vi "Dresden R2R Sputter 03.02.2018 IY24.vi"() -> ()   [LabVIEW 2009]
uses:
  ctl/Roll_StatusT.ctl
  <vilib>/Instr/_visa.llb/VISA Configure Serial Port (Instr).vi
  <vilib>/Utility/file.llb/Read From Spreadsheet File (string).vi
  <vilib>/NI Modbus.llb/MB Serial Master Query Read Discrete Inputs (poly).vi
  <vilib>/NI Modbus.llb/MB Serial Master Query Write Multiple Coils (poly).vi
  <vilib>/NI Modbus.llb/MB Serial Master Query Read Input Registers (poly).vi
  <vilib>/NI Modbus.llb/MB Serial Master Query Write Single Coil (poly).vi
  <vilib>/picture/picture.llb/Draw True-Color Pixmap.vi
panel:
  out "Actual Region led 5":bool
  out "Elapsed Time (s) 10":dbl caption="Elapsed Time (s)"
  in  "Right to Left 5":dbl=100000.0
  out "Elapsed Time (s) 9":dbl caption="Elapsed Time (s)"
  in  "Left to Right 5":dbl=100000.0
  out "Actual Region led 4":bool
  out "Elapsed Time (s) 8":dbl caption="Elapsed Time (s)"
  in  "Right to Left 4":dbl=100000.0
  out "Elapsed Time (s) 7":dbl caption="Elapsed Time (s)"
  in  "Left to Right 4":dbl=100000.0
  out "Actual Region led 3":bool
  out "Elapsed Time (s) 6":dbl caption="Elapsed Time (s)"
  in  "Right to Left 3":dbl=100000.0
  out "Elapsed Time (s) 5":dbl caption="Elapsed Time (s)"
  in  "Left to Right 3":dbl=100000.0
  in  "Speed":dbl=6.85 format="%.2g"
  in  "Roll_side_select":enum32{"Left to Right", "Right to Left"}(radio)=enum."Right to Left"
  in  "Parameters_set":bool
  in  "Calculate_auto":bool
  in  "Test_stop":bool
  in  "Start_roll":bool
  out "COM12 Loop Time":dbl caption="Present (s)" format="%.2f"
  in  "RPM":dbl=13.691
  out "Cevre":dbl
  out "Angle":dbl
  out "Gauge":dbl(knob) min=0.0 max=360.0 step=30.0 scale=0.0..360.0 scale format="%_2f"
  in  "Tension Parametre Set":bool
  out "Bacward Time":dbl
  out "Forward Time":dbl
  in  "Lap Count":i32=1
  in  "Cycle Sayisi":i32=1
  out "Current Chamber":i32=1
  out "Roll Status":T1
  out "Current Forward Lap":i32
  out "Current Cycle":i32
  out "Lap Times":dbl[](array[numeric])
  out "Current Backward Lap":i32
  in  "Moxa I/O 1":refnum<visa-resource-name>=refnum
  in  "Ch1_Motor_DO":bool
  in  "Ch3_Motor_DO":bool
  in  "Ch4_Motor_DO":bool
  in  "Ch2_Motor_DO":bool
  in  "Motor_Dir_DO":bool
  out "Ch1_Sensor_DI":bool
  out "Ch4_Sensor_DI":bool
  out "Ch2_Sensor_DI":bool
  out "Ch3_Sensor_DI":bool
  in  "Sensor_DI Sim":bool
  in  "Sim":bool
  in  "Ch1_3_2_do":bool
  in  "To Right Volt":dbl=6.85 format="%.2g"
  in  "To Left Volt":dbl=6.85 format="%.2g"
  out "COM12 Loop Time":dbl caption="Present (s)" format="%.2f"
  out "COM12 Time":dbl caption="Present (s)" format="%.2f"
  in  "Timer Reset Roll 2":bool
  in  "Left to Right":dbl=100000.0
  out "Elapsed Time (s) 2":dbl caption="Elapsed Time (s)"
  in  "Right to Left":dbl=100000.0
  out "Elapsed Time (s)":dbl
  out "Ch4_tab_led":bool
  out "Ch3_tab_led":bool
  out "Ch2_tab_led":bool
  out "Ch1_tab_led":bool
  in  "Start_Coating_MW":bool
  in  "Statue_abort":bool
  in  "Graph_tab_ch4":enum32{"Page 1"}(tab)
  out "Graph_pumping_time_ch4":dbl caption="Elapsed Time (s)" format="%<%H:%M:%S>t"
  out "Pressure_time_graph_ch4":dbl(graph)
  in  "Graph_tab_ch3":enum32{"Page 1"}(tab)
  out "Graph_pumping_time_ch3":dbl caption="Elapsed Time (s)" format="%<%H:%M:%S>t"
  out "Pressure_time_graph_ch3":dbl(graph)
  in  "Graph_tab_ch2":enum32{"Page 1"}(tab)
  out "Graph_pumping_time_ch2":dbl caption="Elapsed Time (s)" format="%<%H:%M:%S>t"
  out "Pressure_time_graph_ch2":dbl(graph)
  in  "MW_RF_Interlock":dbl=5e-05
  in  "Start_Coating_Ch4":bool
  in  "Single_ch3_Interlock":dbl=5e-05
  in  "MW_Coating_Interlock 6":dbl=5e-05
  in  "Start_Coating_Ch3":bool
  in  "Start_Coating_Ch2":bool
  in  "Single_Ch2_Interlock":dbl=5e-05
  in  "MW_Coating_Interlock 5":dbl=5e-05
  in  "R General_tab":enum32{"Page 1", "Page 2"}(tab)
  in  "R_Cancel":bool caption="Cancel"
  in  "Thickness_Monitor_Active":bool
  in  "Recipe_selection tab":T2(tab)
  in  "R_Simple_Coating Type Selection":T3(radio)
  in  "R_Single_Coating Type Selection_tab":T4(tab)
  in  "R_Single Microwave Time":dbl caption="sec"
  in  "R_Single Microwave Power":dbl caption="Watt"
  in  "R Single Microwave Number":dbl
  in  "R_DC_Chamber_selection":enum32{"Chamber II", "Chamber III"}(radio)
  in  "R Single DC Interval length":dbl
  in  "R Single DC Step5 Coating Power Active":bool
  in  "R Single DC Step5 Coating Power":dbl caption="Watt"
  in  "R Single DC Step4 Coating Power Active":bool
  in  "R Single DC Step4 Coating Power":dbl caption="Watt"
  in  "R Single DC Step3 Coating Power Active":bool
  in  "R Single DC Step3 Coating Power":dbl caption="Watt"
  in  "R Single DC Step2 Coating Power Active":bool
  in  "R Single DC Step2 Coating Power":dbl caption="Watt"
  in  "R Single DC Step1 Coating Power Active":bool
  in  "R Single DC Step1 Coating Power":dbl caption="Watt"
  in  "R_Single DC_Material ok":bool
  in  "R_Single DC_Mat_sel":u64(ring) items=["Other", "Ag", "AgBr", "AgCl", "Al", "Al2O3", "As", "Au", "B", "Ba", "Be", "Bi", "Bi2O3", "C (Diamond)", "C (Graphite)", "Ca", "CaF", "Cd", "CdS", "CdSe", "CdTe", "CeF3", "CeO", "Cr", "Cr2O3", "Co", "Cu", "Cu2S (A)", "Cu2S (B)", "CuS", "Dy", "Er", "Fe", "Ga", "GaAs", "Gd", "Ge", "Hf", "HfO2", "Hg", "Ho", "In", "InSb", "In2O3", "Ir", "KCl", "La", "LaF3", "LaO3", "Li", "LiF", "Mg", "MgF2", "MgO", "Mn", "MnS", "Mo", "Na", "NaCl", "NdF3", "Nd2O3", "Ni", "Nb", "Nb2O5", "Pb", "PbS", "Pd", "Pt", "Re", "Rh", "Rb", "S", "Sb", "Sc", "Se", "Si", "SiO", "SiO2", "Sm", "Sn", "Ta", "Ta2O5", "Te", "Tb", "ThF4", "Ti", "TiO2", "TiO", "Tl", "U", "V", "W", "WC", "Y", "Y2O3", "Yb", "Zn", "ZnO", "ZnSe", "ZnS", "Zr", "ZrO2", "Si3N4", "ITO", "PbI2"]
  in  "R Single DC Target material":string
  in  "R Single DC Ignition Power":dbl caption="Watt"
  in  "R Single DC Target Clean":bool
  in  "R Single DC Target Clean Time":dbl caption="min" format="%.1f"
  in  "R Single DC Target Clean Power":dbl caption="Watt"
  in  "R Single RF Interval length":dbl
  in  "R Single RF Step5 Coating Power Active":bool
  in  "R Single RF Step5 Coating Power":dbl caption="Watt"
  in  "R Single RF Step4 Coating Power Active":bool
  in  "R Single RF Step4 Coating Power":dbl caption="Watt"
  in  "R Single RF Step3 Coating Power Active":bool
  in  "R Single RF Step3 Coating Power":dbl caption="Watt"
  in  "R Single RF Step2 Coating Power Active":bool
  in  "R Single RF Step2 Coating Power":dbl caption="Watt"
  in  "R Single RF Step1 Coating Power Active":bool
  in  "R_Single RF Material ok":bool
  in  "R_Single RF_Mat_sel":u64(ring) items=["Other", "Ag", "AgBr", "AgCl", "Al", "Al2O3", "As", "Au", "B", "Ba", "Be", "Bi", "Bi2O3", "C (Diamond)", "C (Graphite)", "Ca", "CaF", "Cd", "CdS", "CdSe", "CdTe", "CeF3", "CeO", "Cr", "Cr2O3", "Co", "Cu", "Cu2S (A)", "Cu2S (B)", "CuS", "Dy", "Er", "Fe", "Ga", "GaAs", "Gd", "Ge", "Hf", "HfO2", "Hg", "Ho", "In", "InSb", "In2O3", "Ir", "KCl", "La", "LaF3", "LaO3", "Li", "LiF", "Mg", "MgF2", "MgO", "Mn", "MnS", "Mo", "Na", "NaCl", "NdF3", "Nd2O3", "Ni", "Nb", "Nb2O5", "Pb", "PbS", "Pd", "Pt", "Re", "Rh", "Rb", "S", "Sb", "Sc", "Se", "Si", "SiO", "SiO2", "Sm", "Sn", "Ta", "Ta2O5", "Te", "Tb", "ThF4", "Ti", "TiO2", "TiO", "Tl", "U", "V", "W", "WC", "Y", "Y2O3", "Yb", "Zn", "ZnO", "ZnSe", "ZnS", "Zr", "ZrO2", "Si3N4", "ITO", "PbI2"]
  in  "R Single RF Target material":string
  in  "R Single RF Ignition Power":dbl caption="Watt"
  in  "R Single RF Target Clean Power":dbl caption="Watt"
  in  "R Single RF Target Clean Time":dbl caption="min" format="%.1f"
  in  "R Single RF Target Clean":bool
  in  "R Single RF Ramp down":bool
  in  "R Single RF Ramp down Time":dbl caption="sec"
  in  "R Single RF  Step1 Coating Power":dbl caption="Watt"
  in  "R Single RF Ramp up Time":dbl caption="sec"
  in  "R Single RF Ramp up":bool
  in  "R Cmb Interval length":dbl
  in  "R Cmb Ch2 DC Target Clean Power Active":bool
  in  "R Cmb Ch3 Step5 Coating Power":dbl caption="Watt"
  in  "R Cmb Ch3 Step4 Coating Power":dbl caption="Watt"
  in  "R Cmb Ch3 Step3 Coating Power":dbl caption="Watt"
  in  "R Cmb Ch3 Step2 Coating Power":dbl caption="Watt"
  in  "R Cmb Ch3 Step1 Coating Power":dbl caption="Watt"
  in  "R Cmb Ch2 Step5 Coating Power Active":bool
  in  "R Cmb Ch2 Step5 Coating Power":dbl caption="Watt"
  in  "R Cmb Ch2 Step4 Coating Power Active":bool
  in  "R Cmb Ch2 Step4 Coating Power":dbl caption="Watt"
  in  "R Cmb Ch2 Step3 Coating Power Active":bool
  in  "R Cmb Ch2 Step3 Coating Power":dbl caption="Watt"
  in  "R Cmb Ch2 Step2 Coating Power Active":bool
  in  "R Cmb Ch2 Step2 Coating Power":dbl caption="Watt"
  in  "R Cmb Ch2 Step1 Coating Power Active":bool
  in  "R Cmb Ch2 Step1 Coating Power":dbl caption="Watt"
  in  "R Cmb Ch3 Material ok":bool
  in  "R Cmb Ch3 Mat_sel":u64(ring) items=["Other", "Ag", "AgBr", "AgCl", "Al", "Al2O3", "As", "Au", "B", "Ba", "Be", "Bi", "Bi2O3", "C (Diamond)", "C (Graphite)", "Ca", "CaF", "Cd", "CdS", "CdSe", "CdTe", "CeF3", "CeO", "Cr", "Cr2O3", "Co", "Cu", "Cu2S (A)", "Cu2S (B)", "CuS", "Dy", "Er", "Fe", "Ga", "GaAs", "Gd", "Ge", "Hf", "HfO2", "Hg", "Ho", "In", "InSb", "In2O3", "Ir", "KCl", "La", "LaF3", "LaO3", "Li", "LiF", "Mg", "MgF2", "MgO", "Mn", "MnS", "Mo", "Na", "NaCl", "NdF3", "Nd2O3", "Ni", "Nb", "Nb2O5", "Pb", "PbS", "Pd", "Pt", "Re", "Rh", "Rb", "S", "Sb", "Sc", "Se", "Si", "SiO", "SiO2", "Sm", "Sn", "Ta", "Ta2O5", "Te", "Tb", "ThF4", "Ti", "TiO2", "TiO", "Tl", "U", "V", "W", "WC", "Y", "Y2O3", "Yb", "Zn", "ZnO", "ZnSe", "ZnS", "Zr", "ZrO2", "Si3N4", "ITO", "PbI2"]
  in  "R Cmb Ch3 Target material":string
  in  "R Cmb Ch3 DC Ignition Power":dbl caption="Watt"
  in  "R Cmb Ch3 DC Target Clean Power Active":bool
  in  "R Cmb Ch3 DC Target Clean Time":dbl caption="min" format="%.1f"
  in  "R Cmb Ch3 DC Target Clean Power":dbl caption="Watt"
  in  "R_Cmb Ch2_Material ok":bool
  in  "R_Cmb Ch2_Mat_sel":u64(ring) items=["Other", "Ag", "AgBr", "AgCl", "Al", "Al2O3", "As", "Au", "B", "Ba", "Be", "Bi", "Bi2O3", "C (Diamond)", "C (Graphite)", "Ca", "CaF", "Cd", "CdS", "CdSe", "CdTe", "CeF3", "CeO", "Cr", "Cr2O3", "Co", "Cu", "Cu2S (A)", "Cu2S (B)", "CuS", "Dy", "Er", "Fe", "Ga", "GaAs", "Gd", "Ge", "Hf", "HfO2", "Hg", "Ho", "In", "InSb", "In2O3", "Ir", "KCl", "La", "LaF3", "LaO3", "Li", "LiF", "Mg", "MgF2", "MgO", "Mn", "MnS", "Mo", "Na", "NaCl", "NdF3", "Nd2O3", "Ni", "Nb", "Nb2O5", "Pb", "PbS", "Pd", "Pt", "Re", "Rh", "Rb", "S", "Sb", "Sc", "Se", "Si", "SiO", "SiO2", "Sm", "Sn", "Ta", "Ta2O5", "Te", "Tb", "ThF4", "Ti", "TiO2", "TiO", "Tl", "U", "V", "W", "WC", "Y", "Y2O3", "Yb", "Zn", "ZnO", "ZnSe", "ZnS", "Zr", "ZrO2", "Si3N4", "ITO", "PbI2"]
  in  "R Cmb Ch2 Target material":string
  in  "R Cmb Ch2 DC Ignition Power":dbl caption="Watt"
  in  "R Cmb Ch2 DC Target Clean Time":dbl caption="min" format="%.1f"
  in  "R Cmb Ch2 DC Target Clean Power":dbl caption="Watt"
  in  "R Cmb Number of pairs":dbl
  in  "Substrate Material":string
  in  "Recipe Name":string
  in  "R_Recipe_type_selection":enum32{"Single Recipe", "Combination Sputter"}(radio)
  in  "R_Web_selection":enum32{"Web", "Other"}(radio)=enum."Other"
  in  "Web_selection_tab":T5(tab)
  in  "R Web thicness":dbl
  in  "R Maximum diameter":dbl format="%.1f"
  in  "R Minimum diameter":dbl
  in  "R Web speed(cm/min)":dbl
  in  "R Tension Value":dbl
  out "R _Total_length":dbl caption="m" format="%.1f"
  in  "R_Calculate":bool
  in  "R_Thickness Selection":enum32{"Thickness", "Time"}(radio)
  in  "R_Target Thickness Value":dbl format="%.2f"
  in  "R_Duration":dbl caption="%"
  in  "R Set Pressure mtorr":dbl caption="mTorr" format="%.1f"
  in  "R Argon Flow sccm":dbl caption="sccm"
  in  "R Z_factor":dbl format="%_3f"
  in  "R Material_density":dbl caption="g/cm3" format="%_3f"
  in  "R_OK":bool caption="OK2"
  in  "R Toooling_factor":dbl caption="%"
  in  "Clear_error":bool
  in  "Gv_tab_ch2_3_gui":enum32{"Page 1", "Page 2"}(tab)
  in  "Gv_open ch2_3_gui":bool
  in  "Gv_close_ch2_3_gui":bool
  out "Error Message":string
  out "Process_flow":string
  in  "MOUSE":enum32{"Page 1", "Page 2", "Page 3", "Page 4"}(tab)=enum."Page 4"
  out "Mouse Position":cluster{"X":i32, "Y":i32}
  out "Mouse Position 3":cluster{"X":i32, "Y":i32}
  out "Mouse Position 5":cluster{"X":i32, "Y":i32}
  out "Mouse Position 4":cluster{"X":i32, "Y":i32}
  out "Mouse Position 2":cluster{"X":i32, "Y":i32}
  out "Mouse Position 8":cluster{"X":i32, "Y":i32}
  out "Mouse Position 7":cluster{"X":i32, "Y":i32}
  out "Mouse Position 6":cluster{"X":i32, "Y":i32}
  out "Mouse Position 9":cluster{"X":i32, "Y":i32}
  in  "general tab":T6(tab)
  out "DESCRIPTION":string
  in  "Graph_tab_ch1":enum32{"Page 1"}(tab)
  out "Graph_pumping_time_ch1":dbl caption="Elapsed Time (s)" format="%<%H:%M:%S>t"
  out "Pressure_time_graph_ch1":dbl(graph)
  out "Pressure_gui":dbl format="%.1f"
  out "Ch_CC_press_ch1_gui1":dbl format="%#_2e"
  out "Ch_pg_press_ch1_gui":dbl caption="Torr" format="%#_2e"
  out "Pl_pg_press_ch1_gui":dbl caption="Torr" format="%#_2e"
  out "Ch_CC_press_ch2":dbl format="%_2e"
  out "Ch_pg_press_ch2_gui":dbl caption="Torr" format="%#_2e"
  out "Pressure 2_gui":i32 format="%.1f"
  in  "Pl_vbv_ch3_tab_gui":enum32{"Page 1", "Page 2"}(tab)
  in  "Ch3_Pl_vbv_stop_gui":bool
  in  "Ch3_Pl_vbv_start_gui":bool
  in  "Pl_vbv_ch2_tab_gui":enum32{"Page 1", "Page 2"}(tab)
  in  "Ch2_Pl_vbv_stop_gui":bool
  in  "Ch2_Pl_vbv_start_gui":bool
  in  "Mp_ch3_tab_gui":enum32{"Page 1", "Page 2"}(tab)
  in  "Ch3_Mp_stop_gui":bool
  in  "Ch3_Mp_start_gui":bool
  in  "Mp_ch2_tab_gui":enum32{"Page 1", "Page 2"}(tab)
  in  "Ch2_Mp_stop_gui":bool
  in  "Ch2_Mp_start_gui":bool
  in  "Gv_tab_ch1_2_gui":enum32{"Page 1", "Page 2"}(tab)
  in  "Gv_close_ch1_2_gui":bool
  in  "Gv_open ch1_2_gui":bool
  in  "Gv_tab_ch3_4gui":enum32{"Page 1", "Page 2"}(tab)
  in  "Gv_close_ch3_4gui":bool
  in  "Gv_open ch3_4gui":bool
  in  "Pc_bv_tab_ch3_gui":enum32{"Page 1", "Page 2"}(tab)
  in  "Pc_bv_close_ch3_gui":bool
  in  "Pc_bv_open_ch3_gui":bool
  in  "Pc_bv_tab_ch2_gui":enum32{"Page 1", "Page 2"}(tab)
  in  "Pc_bv_close_ch2_gui":bool
  in  "Pc_bv_open_ch2_gui":bool
  in  "Pc_bv_tab_ch4_gui":enum32{"Page 1", "Page 2"}(tab)
  in  "Pc_bv_close_ch4_gui":bool
  in  "Pc_bv_open_ch4_gui":bool
  in  "Pc_bv_tab_ch1_gui":enum32{"Page 1", "Page 2"}(tab)
  in  "Pc_bv_close_ch1_gui":bool
  in  "Pc_bv_open_ch1_gui":bool
  in  "Trns_gv_bp_ch2_gui":enum32{"Page 1", "Page 2"}(tab)
  in  "Ch2_Trns_gv_bp_close_gui":bool
  in  "Ch2_Trns_gv_bp_open_gui":bool
  in  "Trns_gv_bp_ch3_gui":enum32{"Page 1", "Page 2"}(tab)
  in  "Ch3_Trns_gv_bp_close_gui":bool
  in  "Ch3_Trns_gv_bp_open_gui":bool
  in  "Trns_gv_bp2_ch2_gui":enum32{"Page 1", "Page 2"}(tab)
  in  "Ch2_Trns_gv_bp2_close_gui":bool
  in  "Ch2_Trns_gv_bp2_open_gui":bool
  in  "Trns_gv_bp2_ch3_gui":enum32{"Page 1", "Page 2"}(tab)
  in  "Ch3_Trns_gv_bp2_close_gui":bool
  in  "Ch3_Trns_gv_bp2_open_gui":bool
  in  "Tp_ch3_tab_gui":enum32{"Page 1", "Page 2"}(tab)
  in  "Tp_stop_ch3_gui":bool
  in  "Tp_start_ch3_gui":bool
  in  "Tp_ch2_tab_gui":enum32{"Page 1", "Page 2"}(tab)
  in  "Tp_stop_ch2_gui":bool
  in  "Tp_start_ch2_gui":bool
  in  "Tp_ch4_tab_gui":enum32{"Page 1", "Page 2"}(tab)
  in  "Tp_stop_ch4_gui":bool
  in  "Tp_start_ch4_gui":bool
  in  "Tp_ch1_tab_gui":enum32{"Page 1", "Page 2"}(tab)
  in  "Tp_stop_ch1_gui":bool
  in  "Tp_start_ch1_gui":bool
  in  "Ch_vbv_tab_ch3_gui":enum32{"Page 1", "Page 2"}(tab)
  in  "Ch3_Ch_vbv_close_gui":bool
  in  "Ch3_Ch_vbv_open_gui":bool
  in  "Ch_vbv_tab_ch2_gui":enum32{"Page 1", "Page 2"}(tab)
  in  "Ch2_Ch_vbv_close_gui":bool
  in  "Ch2_Ch_vbv_open_gui":bool
  in  "Ch_vbv_tab_ch4_gui":enum32{"Page 1", "Page 2"}(tab)
  in  "Ch4_Ch_vbv_close_gui":bool
  in  "Ch4_Ch_vbv_open_gui":bool
  in  "Ch_vbv_tab_ch1_gui":enum32{"Page 1", "Page 2"}(tab)
  in  "Ch1_Ch_vbv_close_gui":bool
  in  "Ch1_Ch_vbv_open_gui":bool
  in  "Tp_bv_tab_ch3_gui":enum32{"Page 1", "Page 2"}(tab)
  in  "Ch3_Tp_bv_close_gui":bool
  in  "Ch3_Tp_bv_open_gui":bool
  in  "Tp_bv_tab_ch2_gui":enum32{"Page 1", "Page 2"}(tab)
  in  "Ch2_Tp_bv_close_gui":bool
  in  "Ch2_Tp_bv_open_gui":bool
  in  "Tp_bv_tab_ch4_gui":enum32{"Page 1", "Page 2"}(tab)
  in  "Ch4_Tp_bv_close_gui":bool
  in  "Ch4_Tp_bv_open_gui":bool
  in  "Tp_bv_tab_ch1_gui":enum32{"Page 1", "Page 2"}(tab)
  in  "Ch1_Tp_bv_close_gui":bool
  in  "Ch1_Tp_bv_open_gui":bool
  in  "Pl_vbv_tab_ch1_gui":enum32{"Page 1", "Page 2"}(tab)
  in  "Ch1_Pl_vbv_close_gui":bool
  in  "Ch1_Pl_vbv_open_gui":bool
  in  "Pl_vbv_ch4_tab_gui":enum32{"Page 1", "Page 2"}(tab)
  in  "Ch4_Pl_vbv_stop_gui":bool
  in  "Ch4_Pl_vbv_start_gui":bool
  in  "Mp_ch4_tab_gui":enum32{"Page 1", "Page 2"}(tab)
  in  "Ch4_Mp_stop_gui":bool
  in  "Ch4_Mp_start_gui":bool
  in  "Mp_ch1tab_gui":enum32{"Page 1", "Page 2"}(tab)
  ... 2784 more
  # "CHAMBER 4"
  # "CHAMBER 3"
  # "CHAMBER 2"
  # "CHAMBER 1"
  # "Load Coating and Automatic Coating"
  # "Load Coating and Automatic Coating"
  # "Load Coating and Automatic Coating"
  # "PROCESS FLOW"
  # "ERROR MESSAGE"
  # "Chamber Pressure"
  # "Torr"
  # "Automatic Pumping Time"
  # "Chamber Pressure"
  # "Torr"
  # "Automatic Pumping Time"
  # "Chamber Pressure"
  # "Torr"
  # "Automatic Pumping Time"
  # "Coating Interlock :"
  # "Single Coating Interlock            :"
  # "Combination Coating Interlock  :"
  # "Single Coating Interlock             :"
  # "Combination Coating Interlock  :"
  # "Recipe  Selection"
  # "Web  Selection"
  # "Thickness Monitor Parameters"
  # "Pressure Control Parameters"
  # "Material Density       :"
  # "Argon Flow         :"
  # "Z factor                    :"
  # "Set Pressure        :"
  # "Tooling Factor         :"
  # "Coating Type Selction"
  # "Power Value :"
  # "Watt"
  # "Duration      :"
  # "sec"
  # "Times          :"
  # "DCPS Parameters"
  # "Target material          :"
  # "Ignition Power           :"
  # "Target Clean Power    :"
  # "Interval length:"
  # "m"
  # "Coating Power  Step 1:"
  # "Coating Power  Step 2:"
  # "Coating Power  Step 3:"
  # "Coating Power  Step 4:"
  # "Coating Power  Step 5:"
  # "RFPS Parameters"
  # "Target material          :"
  # "Ramp Up Time           :"
  # "Ignition Power           :"
  # "Target Clean Power    :"
  # "Coating Power  Step 1:"
  # "Interval length:"
  # "m"
  # "Coating Power  Step 2:"
  # "Coating Power  Step 3:"
  # "Coating Power  Step 4:"
  # "Coating Power  Step 5:"
  # "Ramp Down Time      :"
  # "DCPS Parameters"
  # "CHAMBER II"
  # "CHAMBER III"
  # "Target material          :"
  # "Target material         :"
  # "Ignition Power           :"
  # "Ignition Power          :"
  # "Target Clean Power    :"
  # "Target Clean Power   :"
  # "Coating Power  Step 1:"
  # "Coating Power  Step 2:"
  # "Coating Power  Step 3:"
  # "Coating Power  Step 4:"
  # "Coating Power  Step 5:"
  # "Interval length:"
  # "m"
  # "Number of pair:"
  # "Roll  Parameters"
  # "Minimum Diameter      :"
  # "mm"
  # "Web Speed              :"
  # "cm / min"
  # "Tension Value         :"
  # "Maximum Diameter     :"
  # "mm"
  # "N"
  # "Web Thickness            :"
  # "µm"
  # "Total Length           :"
  # "Other Parameters"
  # "Thickness Selection         :"
  # "Target Thickness Value   :"
  # "kA"
  # "sec"
  # "Hz"
  # "Hz"
  # "Hz"
  # "Hz"
  # "CH 4"
  # "CH 3"
  # "CH 2"
  # "CH 1"
  # "Torr"
  # "Torr"
  # "Torr"
  # "Torr"
  # "Torr"
  # "mTorr"
  # "mTorr"
  # "mTorr"
  # "mTorr"
  # "mTorr"
  # "DESCRIPTION"
  # "Chamber Pressure"
  # "Torr"
  # "Automatic Pumping Time"
  # "CHAMBER 4"
  # "CHAMBER 2"
  # "CHAMBER 3"
  # "CHAMBER 1"
  # "Valve Control"
  # "Chamber Pressure"
  # "Torr"
  # "Target Pressure"
  # "Torr"
  # "Hour"
  # "Automatic Pumping Time"
  # "TP-BV"
  # "BG-BV"
  # "TRNS -GV-BP"
  # "PC-BV"
  # "Vacuum Pump Control"
  # "Vacuum Break Valve Control"
  # "PL-VBV"
  # "MP"
  # "TP"
  # "CH-VBV"
  # "Turbo Pump Settings"
  # "Low Speed"
  # "Hz"
  # "Tp Status"
  # "P vs t Graph"
  # "Air pressure check"
  # "CH-ATM close"
  # "Chamber Door check"
  # "PL-ATM close"
  # "Center WFS check"
  # "MP start"
  # "WFC  check"
  # "Pipe Line pressure  check"
  # "TRNS-GV close  check"
  # "Chamber pressure  check"
  # "TP stop"
  # "BG-BV  open"
  # "CC close"
  # "Chamber pressure  check"
  # "BG-BV close"
  # "TP  start"
  # "TP-BV close"
  # "Chamber pressure check"
  # "PL-ATM false"
  # "CC  open"
  # "MP stop"
  # "Trns-GV-BP close"
  # "PL-VBV open"
  # "Target Pressure reach"
  # "Pipe Line pressure check"
  # "Automatic  Vacuum Pumping finish"
  # "CH-ATM false"
  # "PC-BV open"
  # "CH-VBV  open"
  # "Trns-GV-BP open/close"
  # "CH-ATM check"
  # "CH-VBV close"
  # "PL-VBV close"
  # "TP-BV open"
  # "Air pressure check"
  # "Chamber Door check"
  # "Center WFS check"
  # "WFC check"
  # "Trns GV close  check"
  # "CH-VBV close"
  # "PL-VBV close"
  # "CH-ATM close"
  # "PL-ATM close"
  # "MP start"
  # "Pipe line pressure  dropped to below 0.9 Torr"
  # "Chamber pressure  dropped to below 0.9 Torr"
  # "TP-BV open"
  # "PC-BV open"
  # "Trns GV-BP  open/close"
  # "Chamber pressure   dropped to below 0.9   Torr"
  # "BG-BV open"
  # "Chamber pressure   dropped to below 0.9   Torr"
  # "TP start"
  # "CC open"
  # "Trns-GV-BP close"
  # "Target Pressure Value reach"
  # "Automatic  Vacuum Pumping finish"
  # "Waiting Tp speed drop to  800 Hz"
  # "CC close"
  # "BG-BV close"
  # "PC-BV close"
  # "PC-BV  open if vacuum break."
  # "TP-BV close"
  # "MP stop"
  # "PL-VBV open"
  # "PL-VBV close"
  # "Waiting Tp speed drop to  730 Hz"
  # "CH-VBV open if vacuum break"
  # "CH-VBV close if vacuum break"
  # "CH-VBV open if vacuum break"
  # "TRNS-GV-BP  open if vacuum break"
  # "CH-ATM check if vacuum break"
  # "TRNS-GV-BP  close"
  # "CH-VBV close if vacuum break"
  # "PC-BV close if vacuum break"
  # "CH-VBV check"
  # "Shutdown process finish"
  # "Vacuum Break Valve Control"
  # "Vacuum Pump Control"
  # "Chamber Pressure"
  # "Torr"
  # "Target Pressure"
  # "Torr"
  # "Hour"
  # "Automatic Pumping Time"
  # "Valve Control"
  # "BG-BV"
  # "TP-BV"
  # "TRNS -GV-BP"
  # "TRNS -GV-BP2"
  # "PC-BV"
  # "TP"
  # "PL-VBV"
  # "MP"
  # "CH-VBV"
  # "Turbo Pump Settings"
  # "Low Speed"
  # "Hz"
  # "Tp Status"
  # "P vs t Graph"
  # "Air pressure check"
  # "TP-BV open"
  # "Chamber Door check"
  # "CH-ATM close"
  # "Center WFS check"
  # "PL-ATM close"
  # "WFC  check"
  # "MP start"
  # "TRNS-GV 2_3_close  check"
  # "Pipe Line pressure  check"
  # "Chamber pressure  check"
  # "TRNS-GV 3_ 4close  check"
  # "TP stop"
  # "BG-BV  open"
  # "Chamber pressure  check"
  # "CC close"
  # "TP  start"
  # "BG-BV close"
  # "TP-BV close"
  # "Chamber pressure check"
  # "PL-ATM false"
  # "CC  open"
  # "Trns-GV-BP close"
  # "MP stop"
  # "Trns-GV-BP2 close"
  # "PL-VBV open"
  # "Target Pressure reach"
  # "Pipe Line pressure check"
  # "CH-ATM false"
  # "Automatic  Vacuum Pumping finish"
  # "PC-BV open"
  # "CH-VBV  open"
  # "Trns-GV-BP2 open/close"
  # "Trns-GV-BP open/close"
  # "CH-ATM check"
  # "CH-VBV close"
  # "PL-VBV close"
  # "Air pressure check"
  # "Chamber Door check"
  # "Center WFS check"
  # "WFC check"
  # "Trns GV_2_3 close  check"
  # "Trns GV_3_4close  check"
  # "CH-VBV close"
  # "PL-VBV close"
  # "CH-ATM close"
  # "PL-ATM close"
  # "MP start"
  # "Pipe line pressure  dropped to below 0.9 Torr"
  # "Chamber pressure  dropped to below 0.9 Torr"
  # "TP-BV open"
  # "PC-BV open"
  # "Trns GV-BP2  open/close"
  # "Trns GV-BP  open/close"
  # "Chamber pressure   dropped to below 0.9   Torr."
  # "BG-BV open"
  # "Chamber pressure   dropped to below 0.9   Torr"
  # "TP2 start"
  # "CC open"
  # "Trns-GV-BP close"
  # "Trns-GV-BP2 close"
  # "Target Pressure Value reach"
  # "Automatic  Vacuum Pumping finish"
  # "Waiting Tp speed drop to  800 Hz"
  # "CC close"
  # "BG-BV close"
  # "PC-BV close"
  # "PC-BV  open if vacuum break."
  # "TP-BV close"
  # "MP stop"
  # "PL-VBV open"
  # "PL-VBV close"
  # "Waiting Tp speed drop to  730 Hz if vacuum break"
  # "CH-VBV open if vacuum break"
  # "CH-VBV close if vacuum break"
  # "CH-VBV open if vacuum break"
  # "TRNS-GV-BP 2 open if vacuum break"
  # "TRNS-GV-BP  open if vacuum break"
  # "CH-ATM check if vacuum break"
  # "TRNS-GV-BP 2 close"
  # "TRNS-GV-BP close"
  # "CH-VBV close if vacuum break"
  # "PC-BV close if vacuum break"
  # "CH-VBV check"
  # "Shutdown process finish"
  # "Valve Control"
  # "Vacuum Break Valve Control"
  # "Vacuum Pump Control"
  # "Chamber Pressure"
  # "Torr"
  # "Target Pressure"
  # "Torr"
  # "Hour"
  # "Automatic Pumping Time"
  # "BG-BV"
  # "TP-BV"
  # "TRNS -GV-BP2"
  # "TRNS -GV-BP"
  # "PC-BV"
  # "TP"
  # "MP"
  # "PL-VBV"
  # "CH-VBV"
  # "Turbo Pump Settings"
  # "Low Speed"
  # "Hz"
  # "Tp Status"
  # "P vs t Graph"
  # "PL-ATM close"
  # "Air pressure check"
  # "MP start"
  # "Chamber Door check"
  # "Pipe Line pressure  check"
  # "Center WFS check"
  # "Chamber pressure  check"
  # "WFC  check"
  # "BG-BV  open"
  # "TRNS-GV 1_2_close  check"
  # "Chamber pressure  check"
  # "TRNS-GV 2_ 3close  check"
  # "TP  start"
  # "TP stop"
  # "Chamber pressure check"
  # "CC close"
  # "CC  open"
  # "BG-BV close"
  # "Trns-GV-BP close"
  # "TP-BV close"
  # "Trns-GV-BP2 close"
  # "PL-ATM false"
  # "Target Pressure reach"
  # "MP stop"
  # "Automatic  Vacuum Pumping finish"
  # "PL-VBV open"
  # "Pipe Line pressure check"
  # "CH-ATM false"
  # "PC-BV open"
  # "CH-VBV  open"
  # "Trns-GV-BP2 open/close"
  # "Trns-GV-BP open/close"
  # "CH-ATM check"
  # "CH-VBV close"
  # "PL-VBV close"
  # "TP-BV open"
  # "CH-ATM close"
  # "Air pressure check"
  # "Chamber Door check"
  # "Center WFS check"
  # "WFC check"
  # "Trns GV close  check"
  # "Trns GV close  check"
  # "CH-VBV close"
  # "PL-VBV close"
  # "CH-ATM close"
  # "PL-ATM close"
  # "MP start"
  # "Pipe line pressure  dropped to below 0.9 Torr"
  # "Chamber pressure  dropped to below 0.9 Torr"
  # "TP-BV open"
  # "PC-BV open"
  # "Trns GV-BP2  open/close"
  # "Trns GV-BP  open/close"
  # "Chamber pressure   dropped to below 0.9   Torr"
  # "BG-BV open"
  # "Chamber pressure   dropped to below 0.9   Torr"
  # "TP2 start"
  # "CC open"
  # "Trns-GV-BP close"
  # "Trns-GV-BP2 close"
  # "Target Pressure Value reach"
  # "Automatic  Vacuum Pumping finish"
  # "Waiting Tp speed drop to  800 Hz"
  # "CC close"
  # "BG-BV close"
  # "PC-BV close"
  # "PC-BV  open if vacuum break."
  # "TP-BV close"
  # "MP stop"
  # "PL-VBV open"
  # "PL-VBV close"
  # "Waiting Tp speed drop to  730 Hz"
  # "CH-VBV open if vacuum break"
  # "CH-VBV close if vacuum break"
  # "CH-VBV open if vacuum break"
  # "TRNS-GV-BP 2 open if vacuum break"
  # "TRNS-GV-BP  open if vacuum break"
  # "CH-ATM check if vacuum break"
  # "TRNS-GV-BP 2 close"
  # "TRNS-GV-BP  close"
  # "CH-VBV close if vacuum break"
  # "PC-BV close if vacuum break"
  # "CH-VBV check"
  # "Shutdown process finish"
  # "Vacuum Break Valve Control"
  # "PL-VBV"
  # "Chamber Pressure"
  # "Torr"
  # "Target Pressure"
  # "Torr"
  # "Hour"
  # "Automatic Pumping Time"
  # "Valve  Control"
  # "TRNS -GV-BP2"
  # "BG-BV"
  # "TP-BV"
  # "PC-BV"
  # "Vacuum Pump Control"
  # "TP"
  # "MP"
  # "CH-VBV"
  # "Turbo Pump Settings"
  # "Low Speed"
  # "Hz"
  # "Tp Status"
  # "P vs t Graph"
  # "Air pressure check"
  # "CH-ATM close"
  # "PL-ATM close"
  # "Chamber Door check"
  # "Center WFS check"
  # "MP start"
  # "Pipe Line pressure  check"
  # "WFC  check"
  # "Chamber pressure  check"
  # "TRNS-GV close  check"
  # "TP stop"
  # "BG-BV  open"
  # "Chamber pressure  check"
  # "CC close"
  # "TP  start"
  # "BG-BV close"
  # "Chamber pressure check"
  # "TP-BV close"
  # "PL-ATM false"
  # "CC  open"
  # "MP stop"
  # "Trns-GV-BP2 close"
  # "Target Pressure reach"
  # "PL-VBV open"
  # "Pipe Line pressure check"
  # "Automatic  Vacuum Pumping finish"
  # "CH-ATM false"
  # "PC-BV open"
  # "CH-VBV  open"
  # "Trns-GV-BP2 open/close"
  # "CH-ATM check"
  # "CH-VBV close"
  # "PL-VBV close"
  # "TP-BV open"
  # "Air pressure check"
  # "Chamber Door check"
  # "Center WFS check"
  # "WFC check"
  # "Trns GV close  check"
  # "CH-VBV1 close"
  # "PL-VBV1 close"
  # "CH-ATM1 close"
  # "PL-ATM1 close"
  # "MP1 start"
  # "Pipe line pressure  dropped to below 0.9 Torr"
  # "Chamber pressure  dropped to below 0.9 Torr"
  # "TP-BV1 open"
  # "PC-BV1 open"
  # "Trns GV-BP2  open/close"
  # "Chamber pressure   dropped to below 0.9   Torr"
  # "BG-BV1 open"
  # "Chamber pressure   dropped to below 0.9   Torr"
  # "TP1 start"
  # "CC open"
  # "Trns-GV-BP2 close"
  # "Target Pressure Value reach"
  # "Automatic  Vacuum Pumping finish"
  # "Waiting Tp speed drop to  800 Hz"
  # "CC close"
  # "BG-BV close"
  # "PC-BV close"
  # "PC-BV  open if vacuum break."
  # "TP-BV close"
  # "MP stop"
  # "PL-VBV open"
  # "PL-VBV close"
  # "Waiting Tp speed drop to  730 Hz"
  # "CH-VBV open if vacuum break"
  # "CH-VBV close if vacuum break"
  # "CH-VBV open if vacuum break"
  # "TRNS-GV-BP  open  if vacuum break"
  # "CH-ATM check if vacuum break"
  # "TRNS-GV-BP  close"
  # "CH-VBV close if vacuum break"
  # "PC-BV close if vacuum break"
  # "CH-VBV check"
  # "Shutdown process finish"
  # "TRANSFER CONTROL"
  # "Present Location"
  # "Target Chamber"
  # "Recipe List"
  # "Load Coating and Automatic Recipe"
  # "Coating Interlock :"
  # "CH1    :"
  # "Minimum Diameter  :"
  # "mm"
  # "Web Speed       :"
  # "cm / min"
  # "Tension Value  :"
  # "Maximum Diameter :"
  # "mm"
  # "N"
  # "Web Thickness        :"
  # "µm"
  # "Target Length"
  # "m"
  # "Target Length"
  # "m"
  # "CST-FIX"
  # "PET-COOL"
  # "SRV-PIST"
  # "BP-BV(R)"
  # "BP-BV(L)"
  # "BP-BV(R)"
  # "BP-BV(L)"
  # "BP-BV(R)"
  # "BP-BV(L)"
  # "Gate Valve Control"
  # "Trns-GV 1-2"
  # "Trns-GV 2-3"
  # "Trns-GV 3-4"
  # "Trns-GV 3-4"
  # "Trns-GV 2-3"
  # "Trns-GV 1-2"
  # "Casette Direction  :"
  # "CH-CC"
  # "GV"
  # "Trns-GV-BP"
  # "Set Value"
  # "Actual Value"
  # "Set Value"
  # "Actual Value"
  # "CC"
  # "TRNS -GV-BP2"
  # "Trns-GV"
  # "CH2"
  # "CH3"
  # "CH4"
  # "PET-COOL"
  # "SRV-PIST"
  # "SRV-PIST"
  # "CST-FIX"
  # "PET-COOL"
  # "CST-FIX"
  # "SRV-PIST"
  # "PET-COOL"
  # "CST-FIX"
  # "CC"
  # "TRNS -GV-BP2"
  # "TRNS -GV-BP"
  # "GV 2-3"
  # "GV 2-1"
  # "CC"
  # "GV 2-3"
  # "TRNS -GV-BP"
  # "TRNS -GV-BP2"
  # "GV 3-4"
  # "Difference between chambers: 1"
  # "Left Direction"
  # "Right Direction"
  # "Casette  transfer 1 -2"
  # "Casette  transfer 2-1"
  # "Casette  transfer 2 -3"
  # "Casette  transfer 3-2"
  # "Casette  transfer 3-4"
  # "Casette transfer 4-3"
  # "Difference between chambers : 2"
  # "Left Direction"
  # "Right Direction"
  # "Casette was transfer  3 to  2"
  # "Casette  transfer 1- 2"
  # "Casette was transfer  2 to  1"
  # "Casette  transfer  2- 3"
  # "Casette was transfer 4 to 3"
  # "Casette  transfer 2 to 3"
  # "Casette was transfer  3 to  2"
  # "Casette  transfer 3 to 4"
  # "Difference between chambers : 3"
  # "Right Direction"
  # "Left Direction"
  # "Casette  transfer  4 to 3"
  # "Casette  transfer 1 to  2"
  # "Casette was transfer  3 to  2"
  # "Casette was transfer  2 to  3"
  # "Casette was transfer 2 to  1"
  # "Casette was transfer  3 to 4"
  # "Transfer Finish"
  # "Start up  Ch1"
  # "Start up Ch2"
  # "GV1-2 open"
  # "GV2-3 CONTROL"
  # "GV3-4 CONTROL"
  # "Right slow deactive"
  # "Right limit deactive"
  # "Left slow active"
  # "Left limit active"
  # "Casette Direction"
  # "Servo-Casette speed set"
  # "Casette Servo Start"
  # "Servo-Casette speed set"
  # "Casette Stop"
  # "Casette Fix Down"
  # "GV Close"
  # "Pet Cool Down"
  # "Srv Pist For"
  # "Deactivation of Sensor"
  # "Transfer Process Finish"
  # "Start up Ch2"
  # "Start up  Ch3"
  # "GV2-3 open"
  # "GV1-2 CONTROL"
  # "GV3-4 CONTROL"
  # "Right slow deactive"
  # "Right limit deactive"
  # "Left slow deactive"
  # "Left limit deactive"
  # "Casette Direction"
  # "Servo-Casette speed set"
  # "Casette Servo Start"
  # "Left Limit&Left Slow Active"
  # "Servo-Casette speed set"
  # "Center Casette Stop"
  # "Casette Fix Down"
  # "GV Close"
  # "Pet Cool Down"
  # "Srv Pist For"
  # "Deactivation of Sensor"
  # "Transfer Process Finish"
  # "Start up  Ch3"
  # "Start up Ch4"
  # "GV3-4open"
  # "GV1-2 CONTROL"
  # "GV2-3 CONTROL"
  # "Right slow deactive"
  # "Right limit deactive"
  # "Left slow deactive"
  # "Left limit deactive"
  # "Casette Direction"
  # "Servo-Casette speed set"
  # "Casette Servo Start"
  # "Left Limit&Left Slow Active"
  # "Servo-Casette speed set"
  # "Center Casette Stop"
  # "Casette Fix Down"
  # "GV Close"
  # "Pet Cool Down"
  # "Srv Pist For"
  # "Deactivation of Sensor"
  # "Transfer Process Finish"
  # "Start up Ch2"
  # "Start up  Ch1"
  # "GV2-1 open"
  # "GV2-3 CONTROL"
  # "GV3-4 CONTROL"
  # "Right slow deactive"
  # "Right limit deactive"
  # "Left slow deactive"
  # "Left limit deactive"
  # "Casette Direction"
  # "Servo-Casette speed set"
  # "Casette Servo Start"
  # "Right Limit&Right Slow Active"
  # "Servo-Casette speed set"
  # "Center Casette Stop"
  # "Casette Fix Down"
  # "GV Close"
  # "Pet Cool Down"
  # "Srv Pist For"
  # "Deactivation of Sensor"
  # "Transfer Process Finish"
  # "Start up Ch3"
  # "Start up  Ch2"
  # "GV2-3open"
  # "GV1-2 CONTROL"
  # "GV3-4 CONTROL"
  # "Right slow deactive"
  # "Right limit deactive"
  # "Left slow deactive"
  # "Left limit deactive"
  # "Casette Direction"
  # "Servo-Casette speed set"
  # "Casette Servo Start"
  # "Right Limit&Right Slow Active"
  # "Servo-Casette speed set"
  # "Center Casette Stop"
  # "Casette Fix Down"
  # "GV Close"
  # "Pet Cool Down"
  # "Srv Pist For"
  # "Deactivation of Sensor"
  # "Transfer Process Finish"
  # "Start up Ch4"
  # "Start up  Ch3"
  # "GV3-4open"
  # "GV1-2 CONTROL"
  # "GV2-3 CONTROL"
  # "Right slow active"
  # "Right limit active"
  # "Left slow deactive"
  # "Left limit deactive"
  # "Casette Direction"
  # "Servo-Casette speed set"
  # "Casette Servo Start"
  # "Servo-Casette speed set"
  # "Center Casette Stop"
  # "Casette Fix Down"
  # "GV Close"
  # "Pet Cool Down"
  # "Srv Pist For"
  # "Deactivation of Sensor"
  # "Transfer Process Finish"
  # "SRV-PIST-BACK-CH1"
  # "SRV-PIST-BACK-CH2"
  # "SRV-PIST-BACK-CH3"
  # "SRV-PIST-BACK-CH4"
  # "PET COOL UP-CH1"
  # "PET COOL UP-CH2"
  # "PET COOL UP-CH3"
  # "PET COOL UP-CH4"
  # "CST FIX UP-CH1"
  # "CST FIX UP-CH2"
  # "CST FIX UP-CH3"
  # "CST FIX UP-CH4"
  # "Routine Check Finish"
  # "TC1 Set Value:"
  # "TC2 Set Value:"
  # "Torr"
  # "Check ZERO Routine"
  # "Transfer"
  # "WATER OPEN"
  # "CC CLOSE"
  # "BG-BV CLOSE"
  # "PC-BV CLOSE"
  # "SOV-Ar Open"
  # "PC-BV OPEN"
  # "CHECK CHAMBER PRESSURE"
  # "PC-BV SET POSITION 10"
  # "CHECK CHAMBER PRESSURE"
  # "SET AR"
  # "CHECK CHAMBER PRESSURE"
  # "Ignite Plasma"
  # "SET PRESSURE"
  # "MW duration"
  # "Microwave Number 1"
  # "Microwave Number 2"
  # "Microwave Number  not equal 1 and 2"
  # "Oscillation pause duration"
  # "Microwave Number  not equal 1 and 2"
  # "Other"
  # "MW CLOSE"
  # "PC-BV OPEN"
  # "SET ZERO Ar FLOW"
  # "SOV Ar Close"
  # "ADD Roll"
  # "CC OPEN"
  # "BG-BV Open"
  # "FINISH"
  # "Transfer"
  # "Check ZERO Routine"
  # "WATER OPEN"
  # "Baratron set zero"
  # "CC CLOSE"
  # "BG-BV OPEN"
  # "CHAMBER PRESSURE AFTER SOV-AR OPEN"
  # "PC-BV CLOSE"
  # "SOV-Ar Open"
  # "CHECK CHAMBER PRESSURE"
  # "CHAMBER PRESSURE before SET Ar"
  # "PC-BV OPEN"
  # "CC OPEN"
  # "CHECK CHAMBER PRESSURE"
  # "CC Close"
  # "SET Ar"
  # "SET PRESSURE"
  # "DC Other-Ignite Plasma"
  # "DC Web- Ignite Plasma"
  # "DC Target Clean Power"
  # "DC-Ignite Plasma Check"
  # "Other Coating"
  # "DC Target Clean Power Process"
  # "Set Pressure"
  # "Change coating power while rolling"
  # "Other"
  # "TM parameters"
  # "Thickness"
  # "Time"
  # "Close DC"
  # "PC-BV Open"
  # "Ar set zero"
  # "Sov-Ar Close"
  # "CC OPEN"
  # "Check Pressure"
  # "Roll Back"
  # "FINISH"
  # "Transfer"
  # "Check ZERO Routine"
  # "WATER OPEN"
  # "BG-BV OPEN"
  # "Baratron set zero"
  # "CC CLOSE"
  # "PC-BV CLOSE"
  # "CHAMBER PRESSURE AFTER SOV-AR OPEN"
  # "SOV-Ar Open"
  # "CHECK CHAMBER PRESSURE"
  # "CHAMBER PRESSURE before SET Ar"
  # "PC-BV OPEN"
  # "CC OPEN"
  # "CHECK CHAMBER PRESSURE"
  # "CC CLOSE"
  # "SET Ar"
  # "SET PRESSURE"
  # "DC-Ignite Plasma"
  # "DC-Ignite Plasma Check"
  # "CHECK CHAMBER PRESSURE"
  # "Other Coating Power"
  # "DC Target Clean Power"
  # "Other Coating Check"
  # "DC Target Clean Power Process"
  # "Set Pressure"
  # "Change coating power while rolling"
  # "Other"
  # "TM parameters"
  # "Thickness"
  # "Time"
  # "Close DC"
  # "PC-BV Open"
  # "Ar set zero"
  # "Sov-Ar Close"
  # "CC Open"
  # "Chamber Pressure Check"
  # "Roll Back"
  # "FINISH"
  # "Check ZERO Routine"
  # "Transfer"
  # "WATER OPEN"
  # "BG-BV OPEN"
  # "Baratron set zero"
  # "CC CLOSE"
  # "CHAMBER PRESSURE AFTER SOV-AR OPEN"
  # "PC-BV CLOSE"
  # "SOV-Ar Open"
  # "CHECK CHAMBER PRESSURE"
  # "CHAMBER PRESSURE before SET Ar"
  # "PC-BV OPEN"
  # "CC OPEN"
  # "CHECK CHAMBER PRESSURE"
  # "CC Close"
  # "SET Ar"
  # "SET PRESSURE"
  # "RF-Ignite Plasma"
  # "RF-Ignite Plasma Check"
  # "Other Coating Power"
  # "CHECK CHAMBER PRESSURE"
  # "Other Coating Power Check"
  # "RF Target Clean Power"
  # "RF Target Clean Power Process"
  # "Change coating power while rolling"
  # "Other"
  # "TM parameters"
  # "Thickness"
  # "Time"
  # "Close RF"
  # "PC-BV Open"
  # "Ar set zero"
  # "Sov-Ar Close"
  # "CC Open"
  # "Chamber Pressure Check"
  # "Roll Back"
  # "FINISH"
  # "Check ZERO Routine"
  # "Transfer"
  # "CH3-WATER FLOW CONTROLLER OPEN"
  # "CH3-CC CLOSE"
  # "CH3-BG-BV CLOSE"
  # "CH3-PC-BV CLOSE"
  # "CH3-SOV-Ar Open"
  # "CH3-PC-BV OPEN"
  # "CH3-CHECK CHAMBER PRESSURE"
  # "SET PRESSURE"
  # "CHECK CHAMBER PRESSURE"
  # "SET Ar Flow"
  # "CHECK CHAMBER PRESSURE"
  # "CH3-DC-Ignite Plasma"
  # "CH3-DC-Ignite Plasma Check"
  # "PC-BV Middle Position"
  # "PC-BV Middle Position"
  # "CH3-DC Target Clean Power"
  # "CH3-DC Target Clean Power Process"
  # "Set Ar Flow"
  # "Set Pressure"
  # "Change coating power while rolling"
  # "Close CH3-DC"
  # "Ar set zero"
  # "CH3-Sov-Ar Close"
  # "CH3-PC-BV Open"
  # "Transfer Ch3 to Ch2"
  # "CH2-WATER FLOW CONTROLLER OPEN"
  # "CH2-CC CLOSE"
  # "CH2-BG-BV CLOSE"
  # "CH2-PC-BV CLOSE"
  # "CH2-SOV-Ar Open"
  # "CH2-PC-BV OPEN"
  # "CHECK CHAMBER PRESSURE"
  # "SET PRESSURE"
  # "CHECK CHAMBER PRESSURE"
  # "SET Ar Flow"
  # "CHECK CHAMBER PRESSURE"
  # "CH2-DC-Ignite Plasma"
  # "CH2-DC-Ignite Plasma Check"
  # "CH2-PC-BV Middle Position"
  # "CH2-PC-BV Middle Position"
  # "CH2-DC Target Clean Power"
  # "CH2-DC Target Clean Power Process"
  # "Set Ar Flow"
  # "Set Pressure"
  # "Change coating power while rolling"
  # "Close CH2-DC"
  # "Ar set zero"
  # "CH2-Sov-Ar Close"
  # "PC-BV Open"
  # "Transfer Ch2 to Ch3"
  # "WATER FLOW CONTROLLER OPEN"
  # "CH3-CC CLOSE"
  # "CH3-BG-BV CLOSE"
  # "CH3-PC-BV CLOSE"
  # "CH3-SOV-Ar Open"
  # "CH3-PC-BV OPEN"
  # "CHECK CHAMBER PRESSURE"
  # "SET PRESSURE"
  # "CHECK CHAMBER PRESSURE"
  # "SET Ar Flow"
  # "CHECK CHAMBER PRESSURE"
  # "CH3-DC-Ignite Plasma"
  # "CH3-DC-Ignite Plasma Check"
  # "CH3-PC-BV Middle Position"
  # "CH3-PC-BV Middle Position"
  # "CH3-DC Target Clean Power"
  # "CH3-DC Target Clean Power Process"
  # "Set Ar Flow"
  # "Set Pressure"
  # "Change coating power while rolling"
  # "Close CH3-DC"
  # "Ar set zero"
  # "CH3-Sov-Ar Close"
  # "CH3-PC-BV Open"
  # "Roll Back"
  # "Press"
  # "Pos"
  # "SYSTEM STATUS"
  # "Torr"
  # "Torr"
  # "mTorr"
  # "Completed Coating Thickness"
  # "%"
  # "Instanteneous Thickness"
  # "kA"
  # "Target Thickness"
  # "kA"
  # "Sputter Process"
  # "Remaining Time    :"
  # "sec"
  # "Target Time          :"
  # "min"
  # "Chamber Pressure:"
  # "Torr"
  # "Pressure Control Parameters"
  # "Argon Flow Controller"
  # "sccm"
  # "Set Value:"
  # "Actual Value :"
  # "sccm"
  # "Pressure Control-Butterfly Valve"
  # "Set position value:"
  # "%"
  # "Actual Position:"
  # "%"
  # "Set pressure value:"
  # "mTorr"
  # "Actual Pressure:"
  # "mTorr"
  # "Thickness Monitor Parameters Control"
  # "Material Density"
  # "Z factor"
  # "Tooling Factor"
  # "Thickness"
  # "Rate"
  # "SOV-Ar"
  # "BG-BV"
  # "PC-BV"
  # "Set Forward Power :"
  # "Watt"
  # "Watt"
  # "Volt"
  # "sec"
  # "sec"
  # "sec"
  # "sec"
  # "CH-CC"
  # "Torr"
  # "mTorr"
  # "Completed Coating Thickness"
  # "%"
  # "Instanteneous Thickness"
  # "kA"
  # "Target Thickness"
  # "kA"
  # "Sputter Process"
  # "Remaining Time    :"
  # "sec"
  # "Target Time          :"
  # "min"
  # "Chamber Pressure:"
  # "Torr"
  # "Pressure Control Parameters"
  # "Argon Flow Controller"
  # "Set Value:"
  # "sccm"
  # "Actual Value :"
  # "sccm"
  # "Pressure Control-Butterfly Valve"
  # "%"
  # "Set position value:"
  # "Position:"
  # "%"
  # "Set pressure value:"
  # "mTorr"
  # "Pressure:"
  # "mTorr"
  # "Thickness Monitor Parameters Control"
  # "Material Density"
  # "Z factor"
  # "Tooling Factor"
  # "Thickness"
  # "Rate"
  # "BG-BV"
  # "PC-BV"
  # "SOV-Ar"
  # "Watt"
  # "Actual DC Power   :"
  # "Watt"
  # "Volt"
  # "Actual DC Potential:"
  # "DC ramp up time :"
  # "sec"
  # "DC ramp down time :"
  # "sec"
  # "CH-CC"
  # "Torr"
  # "mTorr"
  # "Sputter Process"
  # "Remaining Time    :"
  # "sec"
  # "Target Time          :"
  # "min"
  # "Completed Coating Thickness"
  # "%"
  # "Instanteneous Thickness"
  # "kA"
  # "Target Thickness"
  # "kA"
  # "Chamber Pressure:"
  # "Torr"
  # "Pressure Control Parameters"
  # "Argon Flow Controller"
  # "sccm"
  # "Set Value:"
  # "sccm"
  # "Actual Value :"
  # "Pressure Control-Butterfly Valve"
  # "Set position value:"
  # "%"
  # "Position:"
  # "%"
  # "Set pressure value:"
  # "mTorr"
  # "Pressure:"
  # "mTorr"
  # "Thickness Monitor Parameters Control"
  # "Material Density"
  # "Z factor"
  # "Tooling Factor"
  # "Thickness"
  # "Rate"
  # "SOV-Ar"
  # "BG-BV"
  # "PC-BV"
  # "Watt"
  # "Actual DC Power   :"
  # "Watt"
  # "Actual DC Potential:"
  # "Volt"
  # "DC ramp up time :"
  # "sec"
  # "DC ramp down time :"
  # "sec"
  # "CH-CC"
  # "Torr"
  # "mTorr"
  # "Chamber Pressure:"
  # "Torr"
  # "Pressure Control Parameters"
  # "Argon Flow Controller"
  # "sccm"
  # "Set Value:"
  # "Actual Value :"
  # "sccm"
  # "Pressure Control-Butterfly Valve"
  # "Set position value:"
  # "%"
  # "Position:"
  # "%"
  # "Set pressure value:"
  # "mTorr"
  # "Pressure:"
  # "mTorr"
  # "SOV-Ar"
  # "BG-BV"
  # "PC-BV"
  # "Microwave Power Supply Control 1"
  # "Microwave Power Supply Control 2"
  # "Set  Power"
  # "Watt"
  # "Set  Power"
  # "Watt"
  # "CH-CC"